vi "UHR-Fleezers Control (host) - 10.4.vi"() -> ()   [LabVIEW 2010] (continued)
        n1177 = event-data() -> ()  [unwired: 7 out]
        n1178 = Negate(x="Phase adj. (AI1)") -> (-x=w4472:i16)
        n1179 = Select(t=w4472, s="- phase (AI1)", f="Phase adj. (AI1)") -> (s? t:f=w4471:i16)
        n1180 = xnode "Read/Write Control"("FPGA VI Reference In"=w4475, "error in"=w4474, "Phase count adjustment"=w4471) -> ("FPGA VI Reference Out"=w4470:T20, "error out"=w4469:errorcluster)
        n1181 = Or(x="- phase (AI1)", y="+ phase (AI1)") -> (x .or. y?=w4466:bool)
        n1182 = xnode "Read/Write Control"("FPGA VI Reference In"=w4470, "error in"=w4469, "+ phase"=w4466) -> ("error out"=w4465:errorcluster)  [unwired: 1 out]
      }
      event "Signals to Plot": Double Click {
        w4553 = u32 9868950 ("Color Box")
        n1183 = event-data() -> ("Row"=w4555:i32)  [unwired: 9 out]
        n1184 = property on="All Signals" class="WFChart (strict)"("Active Plot"=w4555) -> (error out=w4566:errorcluster)  [unwired: 2 in, 1 out]
        n1185 = property on="All Signals" class="WFChart (strict)" props=["Plot", "Visible?", "Plot", "Plot Color"](error in=w4566) -> (error out=w4565:errorcluster, "Plot.Visible?"=w4564:bool)  [unwired: 1 in, 2 out]
        n1186 = Select(t=FALSE ("Plot.Visible"), s=w4564, f=TRUE ("Plot.Visible")) -> (s? t:f=w4559:bool)
        n1187 = property on="All Signals" class="WFChart (strict)"(error in=w4565, "Plot.Visible?"=w4559) -> (error out=w4561:errorcluster)  [unwired: 1 in, 1 out]
        n1188 = property on="All Signals" class="WFChart (strict)"(error in=w4561) -> (error out=w4556:errorcluster, "Plot.Plot Color"=w4560:u32)  [unwired: 1 in, 1 out]
        n1189 = property on="Signals to Plot" class="LstBox (strict)"(error in=w4556, "Active Row"=w4555) -> (error out=w4554:errorcluster)  [unwired: 1 in, 1 out]
        n1190 = Select(t=w4560, s=w4559, f=u32 0) -> (s? t:f=w4557:u32)
        n1191 = property on="Signals to Plot" class="LstBox (strict)"(error in=w4554, "CellFontColor"=w4557, "SelColor"=w4553, "CellBG"=w4553, "CellFontSize"=u32 20 ("Active Row:Cell Font:Size"), "CellFontBold"=TRUE ("Active Row:Cell Font:Bold")) -> ()  [unwired: 1 in, 2 out]
      }
      event "BD 1 Frequency 1 (MHz)", "BD 1 Frequency 2 (MHz)", "BD 1 Frequency 3 (MHz)", "BD 2 Frequency 1 (MHz)", "BD 2 Frequency 2 (MHz)", "BD 2 Frequency 3 (MHz)", "Trap Delta (MHz)": Value Change {
        # "anytime one of the frequencies is changed, write it to the RF board UNLESS Set 1 is being oscillated. The oscillation\nscript writes the frequencies to the RF board."
        n1192 = event-data() -> ("CtlRef"=w4569:refnum<vi>)  [unwired: 6 out]
        n1193 = control-ref of="Trap Delta (MHz)"() -> (w4568:refnum<vi>)
        n1194 = Equal?(x=w4568, y=w4569) -> (x = y?=w4567:bool)
        n1195 = case shown="False" "Oscillate Set 1" {
          tunnel: w4572 -> [w4592 _]
          tunnel: [w4591 w4595] -> w4571
          tunnel: w4570 -> [w4590 w4595]
          tunnel: w4567 -> [w4575 _]
          frame False {
            n1196 = local read "BD 1 Frequency 2 (MHz)"() -> (w4579:dbl)
            n1197 = local read "BD 1 Frequency 1 (MHz)"() -> (w4577:dbl)
            n1198 = Subtract(x=w4579, y="Trap Delta (MHz)") -> (x-y=w4576:dbl)
            n1199 = Select(t=w4576, s=w4575, f=w4577) -> (s? t:f=w4574:dbl)
            n1200 = local read "Y RF Frequency Limits (MHz)"() -> (w4580:T17)
            n1201 = local read "X RF Frequency Limits (MHz)"() -> (w4581:T17)
            n1202 = local read "BD 1 Frequency 3 (MHz)"() -> (w4593:dbl)
            n1203 = local write "BD 1 Frequency 1 (MHz)"(w4574) -> ()
            n1204 = local read "BD 2 Frequency 1 (MHz)"() -> (w4584:dbl)
            n1205 = local read "BD 2 Frequency 2 (MHz)"() -> (w4583:dbl)
            n1206 = local read "BD 2 Frequency 3 (MHz)"() -> (w4594:dbl)
            n1207 = call "set RF board frequency - interlace.vi"("Board 2 Frequency Limits"=w4580, "Board 1 Frequency Limits"=w4581, "error in"=w4590, "FPGA VI Reference In"=w4592, "Board 2 Frequency 3 (MHz)"=w4594, "Board 1 Frequency 3 (MHz)"=w4593, "Board 2 Frequency 2 (MHz)"=w4583, "Board 2 Frequency 1 (MHz)"=w4584, "Board 1 Frequency 2 (MHz)"=w4579, "Board 1 Frequency 1  (MHz)"=w4574) -> ("error out"=w4591:errorcluster)  [unwired: 1 out]
            n1208 = Subtract(x=w4584, y=w4583) -> (x-y=w4588:dbl)
            n1209 = Subtract(x=w4574, y=w4579) -> (x-y=w4589:dbl)
            n1210 = Square(x=w4588) -> (x^2=w4586:dbl)
            n1211 = Square(x=w4589) -> (x^2=w4587:dbl)
            n1212 = Add(x=w4587, y=w4586) -> (x+y=w4585:dbl)
            n1213 = Square Root(x=w4585) -> (sqrt(x)=w4582:dbl)
            n1214 = local write "Trap Delta (MHz)"(w4582) -> ()
            n1215 = property on="Initial delta (MHz)" class="DigNum (strict)"("Val(Sgnl)"=w4582) -> ()  [unwired: 2 in, 2 out]
          }
          frame True {
          }
        }
      }
      event "Round T1 X": Value Change {
        n1216 = event-data() -> ()  [unwired: 7 out]
        n1217 = local read "BD 1 Frequency 1 (MHz)"() -> (w4598:dbl)
        n1218 = Round To Nearest(number=w4598) -> (nearest integer value=w4597:dbl)
        n1219 = property on="BD 1 Frequency 1 (MHz)" class="DigNum (strict)"("Val(Sgnl)"=w4597) -> ()  [unwired: 2 in, 2 out]
      }
      event "Round T2 X": Value Change {
        n1220 = event-data() -> ()  [unwired: 7 out]
        n1221 = local read "BD 1 Frequency 2 (MHz)"() -> (w4600:dbl)
        n1222 = Round To Nearest(number=w4600) -> (nearest integer value=w4599:dbl)
        n1223 = property on="BD 1 Frequency 2 (MHz)" class="DigNum (strict)"("Val(Sgnl)"=w4599) -> ()  [unwired: 2 in, 2 out]
      }
      event "Stop All": Value Change {
        n1224 = event-data() -> ()  [unwired: 7 out]
        n1225 = local read "Stop All"() -> (w4602:bool)
      }
      event "Delayed Interlace Start": Value Change {
        n1226 = event-data() -> ()  [unwired: 7 out]
        n1227 = flat-sequence {
          frame #0 {
            n1228 = Multiply(x="Delay to Interlace (s)", y=1000.0) -> (x*y=w4605:dbl)
            n1229 = Wait (ms)(milliseconds to wait=w4605) -> ()  [unwired: 1 out]
          }
          frame #1 {
            n1230 = property on="Green laser mode" class="RadioBtnsControl (strict)"("Val(Sgnl)"=enum32{"Laser ON", "Laser OFF", "Interlace"}."Interlace" ("Value (Signaling)")) -> ()  [unwired: 2 in, 2 out]
          }
        }
      }
      event "BD 1 Amplitude 1 (%)", "BD 1 Amplitude 2 (%)", "BD 1 Amplitude 3 (%)", "BD 2 Amplitude 1 (%)", "BD 2 Amplitude 2 (%)", "BD 2 Amplitude 3 (%)", "Trap 1 ON", "Trap 2 ON", "Trap 3 ON", "Feedback On/Off", "All FB On/Off": Value Change {
        w4629 = i16 1 ("f")
        n1231 = event-data() -> ()  [unwired: 7 out]
        n1232 = local write "Trap 1 (ON/OFF)"("Trap 1 ON") -> ()
        n1233 = local write "Trap 2 (ON/OFF)"("Trap 2 ON") -> ()
        n1234 = Boolean To (0,1)(Boolean="Trap 3 ON") -> (0, 1=w4630:i16)
        n1235 = Boolean To (0,1)(Boolean="Trap 1 ON") -> (0, 1=w4631:i16)
        n1236 = Boolean To (0,1)(Boolean="Trap 2 ON") -> (0, 1=w4632:i16)
        n1237 = Select(t=w4632, s="Trap ON/OFF X or Y Amp?", f=w4629) -> (s? t:f=w4627:i16)
        n1238 = Select(t=w4631, s="Trap ON/OFF X or Y Amp?", f=w4629) -> (s? t:f=w4628:i16)
        n1239 = Select(t=w4630, s="Trap ON/OFF X or Y Amp?", f=w4629) -> (s? t:f=w4626:i16)
        n1240 = Select(t=w4629, s="Trap ON/OFF X or Y Amp?", f=w4632) -> (s? t:f=w4624:i16)
        n1241 = Select(t=w4629, s="Trap ON/OFF X or Y Amp?", f=w4631) -> (s? t:f=w4625:i16)
        n1242 = Select(t=w4629, s="Trap ON/OFF X or Y Amp?", f=w4630) -> (s? t:f=w4623:i16)
        n1243 = And(x="All FB On/Off", y="Feedback On/Off") -> (x .and. y?=w4621:cluster{"Set 1":bool, "Set 2":bool})
        n1244 = local read "BD 1 Amplitude 1 (%)"() -> (w4641:dbl)
        n1245 = local read "BD 1 Amplitude 2 (%)"() -> (w4640:dbl)
        n1246 = local read "BD 1 Amplitude 3 (%)"() -> (w4639:dbl)
        n1247 = Unbundle By Name(w4621) -> ("Set 1"=w4616:bool, "Set 2"=w4613:bool)
        n1248 = local read "Y RF Amplitude Limits (%)"() -> (w4609:T17)
        n1249 = local read "X RF Amplitude Limits (%)"() -> (w4610:T17)
        n1250 = local read "BD 2 Amplitude 1 (%)"() -> (w4642:dbl)
        n1251 = local read "BD 2 Amplitude 2 (%)"() -> (w4643:dbl)
        n1252 = local read "BD 2 Amplitude 3 (%)"() -> (w4644:dbl)
        n1253 = And(x="Trap 2 ON", y=w4613) -> (x .and. y?=w4611:bool)
        n1254 = And(x="Trap 1 ON", y=w4616) -> (x .and. y?=w4614:bool)
        n1255 = Multiply(x=w4628, y=w4641) -> (x*y=w4636:dbl)
        n1256 = Multiply(x=w4640, y=w4627) -> (x*y=w4634:dbl)
        n1257 = Multiply(x=w4639, y=w4626) -> (x*y=w4635:dbl)
        n1258 = Multiply(x=w4642, y=w4625) -> (x*y=w4645:dbl)
        n1259 = Multiply(x=w4643, y=w4624) -> (x*y=w4646:dbl)
        n1260 = Multiply(x=w4644, y=w4623) -> (x*y=w4647:dbl)
        n1261 = call "set RF board amplitude - interlace.vi"("Board 2 Amplitude Limits"=w4609, "Board 1 Amplitude Limits"=w4610, "error in"=w4637, "FPGA VI Reference In"=w4638, "Board 2 Amplitude 3 (%)"=w4647, "Board 1 Amplitude 3 (%)"=w4635, "Board 2 Amplitude 2 (%)"=w4646, "Board 2 Amplitude 1 (%)"=w4645, "Board 1 Amplitude 2 (%)"=w4634, "Board 1 Amplitude 1 (%)"=w4636) -> ("error out"=w4618:errorcluster, "FPGA VI Reference Out"=w4619:T20)
        n1262 = xnode "Read/Write Control"("FPGA VI Reference In"=w4619, "error in"=w4618, "FB On/Off Set 1"=w4614, "FB On/Off Set 2"=w4611) -> ("error out"=w4617:errorcluster)  [unwired: 1 out]
      }
      event "Load parameters": Value Change {
        n1263 = event-data() -> ()  [unwired: 7 out]
        n1264 = property on="Saved AOD Raster Scan Parameter Sets" class="Arr (strict)"() -> ("Index Values"=w4717:u32[])  [unwired: 2 in, 2 out]
        n1265 = Index Array(array=w4717, index=0) -> (element=w4714:u32)
        n1266 = local write "Load parameters"(FALSE ("Load parameters")) -> ()
        n1267 = Index Array(array="Saved AOD Raster Scan Parameter Sets", index=w4714) -> (element=w4713:T46)
        n1268 = Unbundle By Name(w4713) -> ("Scan Range AOD (nm) 2"=w4712:dbl, "Step Size AOD (nm) 2"=w4711:dbl, "Scan Speed AOD (nm/s) 2"=w4710:dbl, "Number of scans (AOD) 2"=w4709:u16)
        n1269 = flat-sequence {
          tunnel: w4712 -> [w4720]
          tunnel: w4711 -> [w4719]
          tunnel: w4710 -> [w4718]
          tunnel: w4709 -> [w4721]
          frame #0 {
            n1270 = local write "Scan Speed (nm/s)"(w4718) -> ()
            n1271 = local write "Scan Range (nm)"(w4720) -> ()
            n1272 = local write "Step Size (nm)"(w4719) -> ()
          }
          frame #1 {
            n1273 = property on="Number of F/B Scans (AOD)" class="DigNum (strict)"("Val(Sgnl)"=w4721) -> ()  [unwired: 2 in, 2 out]
          }
        }
      }
      event "Trap 1 (ON/OFF)", "Trap 2 (ON/OFF)": Value Change {
        n1274 = event-data() -> ()  [unwired: 7 out]
        n1275 = property on="Trap 2 ON" class="Bool (strict)"("Val(Sgnl)"="Trap 2 (ON/OFF)") -> ()  [unwired: 2 in, 2 out]
        n1276 = property on="Trap 1 ON" class="Bool (strict)"("Val(Sgnl)"="Trap 1 (ON/OFF)") -> ()  [unwired: 2 in, 2 out]
      }
      event "DIO count 1 (ticks)", "DIO count 2 (ticks)", "DIO count 3 (ticks)", "Interlace", "Number Interlace Sets", "Not-Interlacing Set": Value Change {
        n1277 = event-data() -> ()  [unwired: 7 out]
        n1278 = local read "DIO count 3 (ticks)"() -> (w4734:u32)
        n1279 = local read "DIO count 1 (ticks)"() -> (w4736:u32)
        n1280 = local read "DIO count 2 (ticks)"() -> (w4735:u32)
        n1281 = To Unsigned Byte Integer(number="Not-Interlacing Set") -> (unsigned 8bit integer=w4725:u8)
        n1282 = Add(x=w4725, y=u8 1) -> (x+y=w4729:u8)
        n1283 = xnode "Read/Write Control"("FPGA VI Reference In"=w4740, "error in"=w4738, "DIO count 1 (ticks)"=w4736, "DIO count 2 (ticks)"=w4735, "DIO count 3 (ticks)"=w4734, "Interlace ON/OFF"="Interlace", "Number Interlace Cycles"="Number Interlace Sets", "Interlace Off Parameters"=w4729) -> ("error out"=w4739:errorcluster)  [unwired: 1 out]
        n1284 = Build Array(w4736, w4735, w4734) -> (w4727:u32[])
        n1285 = Split 1D Array(array=w4727, index="Number Interlace Sets") -> (first subarray=w4737:u32[])  [unwired: 1 out]
        n1286 = Index Array(array=w4727, index=w4725) -> (element=w4726:u32)
        n1287 = Add Array Elements(numeric array=w4737) -> (sum=w4731:u32)
        n1288 = Select(t=w4731, s="Interlace", f=w4726) -> (s? t:f=→"Total Counts (ticks)":u32)
      }
      event "Reset Feedback": Value Change {
        n1289 = event-data() -> ()  [unwired: 7 out]
        n1290 = Unbundle By Name("Reset Feedback") -> ("Set 1"=w4882:bool, "Set 2"=w4881:bool)
        n1291 = xnode "Read/Write Control"("FPGA VI Reference In"=w4884, "error in"=w4879, "FB Reset Set 1"=w4882, "FB Reset Set 2"=w4881) -> ("error out"=w4880:errorcluster)  [unwired: 1 out]
      }
      event "PID Gains": Value Change {
        n1292 = event-data() -> ()  [unwired: 7 out]
        n1293 = Unbundle By Name("PID Gains") -> ("Set 1"=w4947:T15, "Set 2"=w4946:T15)
        n1294 = xnode "Read/Write Control"("FPGA VI Reference In"=w4948, "error in"=w4944, "FB Gains Set 1"=w4947, "FB Gains Set 2"=w4946) -> ("error out"=w4945:errorcluster)  [unwired: 1 out]
      }
      event "AI2 to Setpoint", "Setpoints (V)": Value Change {
        n1295 = event-data() -> ()  [unwired: 7 out]
        n1296 = xnode "Read/Write Control"("FPGA VI Reference In"=w5023, "error in"=w5019) -> ("FPGA VI Reference Out"=w5022:T20, "error out"=w5021:errorcluster, "AI2 Y Sum Set 1"=w5030:i16, "AI2 Y Sum Set 2"=w5029:i16)
        n1297 = Cluster To Array(cluster="AI2 to Setpoint") -> (array=w5033:bool[])
        n1298 = local read "AI2 (V)"() -> (w5031:cluster{"Set 1":dbl, "Set 2":dbl})
        n1299 = Or Array Elements(Boolean array=w5033) -> (logical OR=w5034:bool)
        n1300 = Bundle By Name(cluster=w5031, "Set 1"=w5030, "Set 2"=w5029) -> (w5028:cluster{"Set 1":dbl, "Set 2":dbl})
        n1301 = Divide(x=w5028, y=3276.7) -> (x/y=w5027:cluster{"Set 1":dbl, "Set 2":dbl})
        "AI2 (V)" <- w5027
        n1302 = case shown="True" w5034 {
          tunnel: [w5098 w5115] -> w5026
          tunnel: "AI2 to Setpoint" -> [_ w5111]
          tunnel: "Setpoints (V)" -> [w5099 w5114]
          tunnel: w5027 -> [_ w5108]
          frame False {
            n1303 = Multiply(x=3276.7, y=w5099) -> (x*y=w5100:cluster{"Set 1":dbl, "Set 2":dbl})
            n1304 = To Word Integer(number=w5100) -> (16bit integer=w5098:cluster{"Set 1":i16, "Set 2":i16})
          }
          frame True {
            n1305 = Unbundle By Name(w5108) -> ("Set 1"=w5107:dbl, "Set 2"=w5106:dbl)
            n1306 = Unbundle By Name(w5114) -> ("Set 1"=w5113:dbl, "Set 2"=w5112:dbl)
            n1307 = Unbundle By Name(w5111) -> ("Set 1"=w5110:bool, "Set 2"=w5109:bool)
            n1308 = Select(t=w5107, s=w5110, f=w5113) -> (s? t:f=w5105:dbl)
            n1309 = Select(t=w5106, s=w5109, f=w5112) -> (s? t:f=w5104:dbl)
            n1310 = Bundle By Name(cluster=w5114, "Set 1"=w5105, "Set 2"=w5104) -> (w5102:cluster{"Set 1":dbl, "Set 2":dbl})
            n1311 = local write "Setpoints (V)"(w5102) -> ()
            n1312 = Multiply(x=3276.7, y=w5102) -> (x*y=w5103:cluster{"Set 1":dbl, "Set 2":dbl})
            n1313 = To Word Integer(number=w5103) -> (16bit integer=w5115:cluster{"Set 1":i16, "Set 2":i16})
          }
        }
        n1314 = Unbundle By Name(w5026) -> ("Set 1"=w5025:i16, "Set 2"=w5024:i16)
        n1315 = xnode "Read/Write Control"("FPGA VI Reference In"=w5022, "error in"=w5021, "FB Setpoint Set 1"=w5025, "FB Setpoint Set 2"=w5024) -> ("error out"=w5020:errorcluster)  [unwired: 1 out]
      }
      event "Invert GI": Value Change {
        n1316 = event-data() -> ()  [unwired: 7 out]
        n1317 = xnode "Read/Write Control"("FPGA VI Reference In"=w5177, "error in"=w5175, "Invert GI"="Invert GI", "Invert GI 2"="Invert GI") -> ("error out"=w5176:errorcluster)  [unwired: 1 out]
      }
      event "Green FB Setpoint (mV)", "Green FB Gains", "Green FB On/Off", "Current When FB OFF (%)", "Green int current ON count adj": Value Change {
        n1318 = event-data() -> ()  [unwired: 7 out]
        n1319 = local read "Green FB Setpoint (mV)"() -> (w5243:dbl)
        n1320 = local read "Current When FB OFF (%)"() -> (w5246:dbl)
        n1321 = Multiply(x=w5243, y=3.2767) -> (x*y=w5242:dbl)
        n1322 = Multiply(x=w5246, y=655.35) -> (x*y=w5247:dbl)
        n1323 = To Unsigned Word Integer(number=w5247) -> (unsigned 16bit integer=w5245:u16)
        n1324 = local read "Green int current ON count adj"() -> (w5250:u32)
        n1325 = local read "Green FB Gains"() -> (w5249:T15)
        n1326 = local read "Green Laser ON/Interlacing"() -> (w5240:bool)
        n1327 = local read "Green laser mode"() -> (w5239:enum32{"Laser ON", "Laser OFF", "Interlace"})
        n1328 = local read "Green FB On/Off"() -> (w5251:bool)
        n1329 = Equal?(x=w5239, y=enum32{"Laser ON", "Laser OFF", "Interlace"}."Interlace") -> (x = y?=w5237:bool)
        n1330 = Compound Arithmetic op=AND(w5237, w5251, w5240) -> (w5241:bool)
        n1331 = xnode "Read/Write Control"("FPGA VI Reference In"=w5254, "error in"=w5253, "Green FB Setpoint"=w5242, "Green FB On/Off"=w5241, "Current Out"=w5245, "Green int current ON count adj"=w5250, "Green FB Gains"=w5249) -> ("error out"=w5252:errorcluster)  [unwired: 1 out]
      }
      event "Green laser mode", "Green Laser ON/Interlacing": Value Change {
        n1332 = event-data() -> ()  [unwired: 7 out]
        n1333 = case shown="True" "Green Laser ON/Interlacing" {
          tunnel: "Green laser mode" -> [_ w5392]
          tunnel: [enum32{"Laser ON", "Laser OFF", "Interlace"}."Laser OFF" ("Green laser mode") w5392] -> w5380
          tunnel: [FALSE w5388] -> w5379
          frame False {
          }
          frame True {
            n1334 = local read "Green FB On/Off"() -> (w5389:bool)
            n1335 = Equal?(x=w5392, y=enum32{"Laser ON", "Laser OFF", "Interlace"}."Interlace") -> (x = y?=w5390:bool)
            n1336 = And(x=w5390, y=w5389) -> (x .and. y?=w5388:bool)
          }
        }
        n1337 = xnode "Read/Write Control"("FPGA VI Reference In"=w5385, "error in"=w5383, "Operating Mode"=w5380, "Operating Mode 2"=w5380, "Green FB On/Off"=w5379) -> ("error out"=w5384:errorcluster)  [unwired: 1 out]
      }
      event "- phase (APD 1 Gate)", "+ phase (APD 1 Gate)": Value Change {
        n1338 = event-data() -> ()  [unwired: 7 out]
        n1339 = local read "Phase Adj. (APD 1 Gate)"() -> (w5471:i16)
        n1340 = Negate(x=w5471) -> (-x=w5479:i16)
        n1341 = Select(t=w5479, s="- phase (APD 1 Gate)", f=w5471) -> (s? t:f=w5478:i16)
        n1342 = Or(x="- phase (APD 1 Gate)", y="+ phase (APD 1 Gate)") -> (x .or. y?=w5474:bool)
        n1343 = xnode "Read/Write Control"("FPGA VI Reference In"=w5481, "error in"=w5480, "Phase count adjustment (APD 1 Gate)"=w5478) -> ("FPGA VI Reference Out"=w5476:T20, "error out"=w5477:errorcluster)
        n1344 = xnode "Read/Write Control"("FPGA VI Reference In"=w5476, "error in"=w5477, "+ phase (APD 1 Gate)"=w5474) -> ("error out"=w5475:errorcluster)  [unwired: 1 out]
      }
      event "+ phase (APD 2 Gate)", "- phase (APD 2 Gate)": Value Change {
        n1345 = event-data() -> ()  [unwired: 7 out]
        n1346 = local read "Phase Adj. (APD 2 Gate)"() -> (w5557:i16)
        n1347 = Negate(x=w5557) -> (-x=w5565:i16)
        n1348 = Select(t=w5565, s="- phase (APD 2 Gate)", f=w5557) -> (s? t:f=w5564:i16)
        n1349 = Or(x="- phase (APD 2 Gate)", y="+ phase (APD 2 Gate)") -> (x .or. y?=w5560:bool)
        n1350 = xnode "Read/Write Control"("FPGA VI Reference In"=w5567, "error in"=w5566, "Phase count adjustment (APD 2 Gate)"=w5564) -> ("FPGA VI Reference Out"=w5562:T20, "error out"=w5563:errorcluster)
        n1351 = xnode "Read/Write Control"("FPGA VI Reference In"=w5562, "error in"=w5563, "+ phase (APD 2 Gate)"=w5560) -> ("error out"=w5561:errorcluster)  [unwired: 1 out]
      }
      event "Phase Adj. (APD Acq)", "+ phase (APD Acq)", "- phase (APD Acq)": Value Change {
        n1352 = event-data() -> ()  [unwired: 7 out]
        n1353 = local read "Phase Adj. (APD Acq)"() -> (w5645:i16)
        n1354 = Negate(x=w5645) -> (-x=w5651:i16)
        n1355 = Select(t=w5651, s="+ phase (APD Acq)", f=w5645) -> (s? t:f=w5650:i16)
        n1356 = Or(x="+ phase (APD Acq)", y="- phase (APD Acq)") -> (x .or. y?=w5646:bool)
        n1357 = xnode "Read/Write Control"("FPGA VI Reference In"=w5653, "error in"=w5652, "Phase Count Adjustment (APD Acq)"=w5650) -> ("FPGA VI Reference Out"=w5648:T20, "error out"=w5649:errorcluster)
        n1358 = xnode "Read/Write Control"("FPGA VI Reference In"=w5648, "error in"=w5649, "+ phase (APD Acq)"=w5646) -> ("error out"=w5647:errorcluster)  [unwired: 1 out]
      }
      event "Phase adj. (GI)", "+ phase (GI)", "- phase (GI)": Value Change {
        n1359 = event-data() -> ()  [unwired: 7 out]
        n1360 = Negate(x="Phase adj. (GI)") -> (-x=w5737:i16)
        n1361 = Select(t=w5737, s="+ phase (GI)", f="Phase adj. (GI)") -> (s? t:f=w5736:i16)
        n1362 = Or(x="+ phase (GI)", y="- phase (GI)") -> (x .or. y?=w5732:bool)
        n1363 = xnode "Read/Write Control"("FPGA VI Reference In"=w5739, "error in"=w5738, "Phase count adjustment (GI)"=w5736) -> ("FPGA VI Reference Out"=w5734:T20, "error out"=w5735:errorcluster)
        n1364 = xnode "Read/Write Control"("FPGA VI Reference In"=w5734, "error in"=w5735, "+ phase (GI)"=w5732) -> ("error out"=w5733:errorcluster)  [unwired: 1 out]
      }
      event "Phase adj. (GI) 2", "+ phase (GI) 2", "- phase (GI) 2": Value Change {
        n1365 = event-data() -> ()  [unwired: 7 out]
        n1366 = Negate(x="Phase adj. (GI) 2") -> (-x=w5823:i16)
        n1367 = Select(t=w5823, s="+ phase (GI) 2", f="Phase adj. (GI) 2") -> (s? t:f=w5822:i16)
        n1368 = Or(x="+ phase (GI) 2", y="- phase (GI) 2") -> (x .or. y?=w5818:bool)
        n1369 = xnode "Read/Write Control"("FPGA VI Reference In"=w5825, "error in"=w5824, "Phase count adjustment (GI) 2"=w5822) -> ("FPGA VI Reference Out"=w5820:T20, "error out"=w5821:errorcluster)
        n1370 = xnode "Read/Write Control"("FPGA VI Reference In"=w5820, "error in"=w5821, "+ phase (GI) 2"=w5818) -> ("error out"=w5819:errorcluster)  [unwired: 1 out]
      }
      event "Phase adj. (Green FB)", "- phase (Green FB)", "+ phase (Green FB)": Value Change {
        n1371 = event-data() -> ()  [unwired: 7 out]
        n1372 = Negate(x="Phase adj. (Green FB)") -> (-x=w5909:i16)
        n1373 = Select(t=w5909, s="+ phase (Green FB)", f="Phase adj. (Green FB)") -> (s? t:f=w5908:i16)
        n1374 = Or(x="+ phase (Green FB)", y="- phase (Green FB)") -> (x .or. y?=w5904:bool)
        n1375 = xnode "Read/Write Control"("FPGA VI Reference In"=w5911, "error in"=w5910, "Phase count adjustment (Green FB)"=w5908) -> ("FPGA VI Reference Out"=w5906:T20, "error out"=w5907:errorcluster)
        n1376 = xnode "Read/Write Control"("FPGA VI Reference In"=w5906, "error in"=w5907, "+ phase (Green FB)"=w5904) -> ("error out"=w5905:errorcluster)  [unwired: 1 out]
      }
      event "Invert APD Gate", "APD Gate ON Count", "APD Gate OFF Count", "APD Gate", "APD Integration Time (s)", "APD 1 AO Mult.", "APD 2 AO Mult.": Value Change {
        n1377 = event-data() -> ()  [unwired: 7 out]
        n1378 = local read "APD Integration Time (s)"() -> (w5987:dbl)
        n1379 = local read "APD Gate ON Count"() -> (w6000:u32)
        n1380 = local read "APD Gate OFF Count"() -> (w5999:u32)
        n1381 = local read "Invert APD Gate"() -> (w6001:bool)
        n1382 = local read "APD Gate"() -> (w5998:enum32{"ON", "OFF", "Interlace"})
        n1383 = Multiply(x=w5987, y=40000000.0) -> (x*y=w5996:dbl)
        n1384 = Reciprocal(x=w5987) -> (1/x=→"APD Acq Rate (Hz)":dbl)
        n1385 = To Unsigned Long Integer(number=w5996) -> (unsigned 32bit integer=w5995:u32)
        n1386 = local read "DMA Update Period (s)"() -> (w5988:dbl)
        n1387 = Divide(x=w5988, y=w5987) -> (x/y=w5991:dbl)
        n1388 = local read "APD 1 AO Mult."() -> (w5993:i16)
        n1389 = local read "APD 2 AO Mult."() -> (w5992:i16)
        n1390 = Multiply(x=2.0, y=w5991) -> (x*y=w5990:dbl)
        n1391 = local write "APD Samples/FIFO Acq."(w5991) -> ()
        n1392 = local write "APD Elements/DMA read"(w5990) -> ()
        n1393 = xnode "Read/Write Control"("FPGA VI Reference In"=w6004, "error in"=w6003, "Invert APD Gate"=w6001, "APD Gate ON Count"=w6000, "APD Gate OFF Count"=w5999, "APD Acq Rate Count"=w5995, "APD Gate Operating Mode"=w5998, "APD 1 AO scale factor"=w5993, "APD 2 AO scale factor"=w5992) -> ("error out"=w6002:errorcluster)  [unwired: 1 out]
      }
      event "GI Frequency, ON count", "Green FB Count", "GI Frequency, OFF count": Value Change {
        n1394 = event-data() -> ()  [unwired: 7 out]
        n1395 = xnode "Read/Write Control"("FPGA VI Reference In"=w6168, "error in"=w6166, "Green interlace ON count"="GI Frequency, ON count", "Green interlace OFF count"="GI Frequency, OFF count", "Green interlace ON count 2"="GI Frequency, ON count", "Green interlace OFF count 2"="GI Frequency, OFF count", "Green FB Count"="Green FB Count") -> ("error out"=w6167:errorcluster)  [unwired: 1 out]
      }
      event "Number of F/B Scans (AOD)", "Scan Speed (nm/s)", "Scan BD", "Initial delta (MHz)", "Step Size (nm)", "Scan Range (nm)": Value Change {
        w6347 = 123.0  # AOM cal (nm/MHz)
        n1396 = event-data() -> ()  [unwired: 7 out]
        n1397 = local read "BD 1 Frequency 1 (MHz)"() -> (w6330:dbl)
        n1398 = local read "AOM X Cal (nm/MHz)"() -> (w6322:dbl)
        n1399 = local read "X RF Frequency Limits (MHz)"() -> (w6334:T17)
        n1400 = local read "Y RF Frequency Limits (MHz)"() -> (w6331:T17)
        n1401 = local read "BD 2 Frequency 1 (MHz)"() -> (w6336:dbl)
        n1402 = Negate(x="Scan Range (nm)") -> (-x=w6300:dbl)
        n1403 = Divide(x=w6300, y=w6322) -> (x/y=w6304:dbl)
        n1404 = Select(t=w6334, s="Scan BD", f=w6331) -> (s? t:f=w6333:T17)
        n1405 = Select(t=w6330, s="Scan BD", f=w6336) -> (s? t:f=w6335:dbl)
        n1406 = Unbundle By Name(w6333) -> ("Maximum"=w6342:dbl, "Minimum"=w6341:dbl)
        n1407 = Add(x=w6304, y=w6335) -> (x+y=w6339:dbl)
        n1408 = Divide(x=w6300, y="Step Size (nm)") -> (x/y=w6319:dbl)
        n1409 = Divide(x="Step Size (nm)", y=w6322) -> (x/y=w6328:dbl)
        n1410 = Absolute Value(x=w6319) -> (abs(x)=w6303:dbl)
        n1411 = Sign(1:w6300) -> (0:w6301:dbl)
        n1412 = In Range and Coerce(upper limit=w6342, x=w6339, lower limit=w6341) -> (coerced(x)=w6338:dbl, In Range?=w6340:bool)
        n1413 = To Unsigned Quad Integer(1:w6303) -> (0:w6318:u64)
        "Scan steps (AOD)" <- w6318
        n1414 = call "IR AOM freq to word.vi"("Frequency In (MHz)"=w6328) -> ("Frequency Word Out (double)"=w6325:dbl)
        n1415 = Multiply(x=w6301, y=w6325) -> (x*y=w6302:dbl)
        n1416 = Subtract(x=w6339, y=w6338) -> (x-y=w6337:dbl)
        n1417 = To Quad Integer(1:w6302) -> (0:w6324:i64)
        "Incr. int (AOD)" <- w6324
        n1418 = Subtract(x=w6304, y=w6337) -> (x-y=w6323:dbl)
        "Scan Range (MHz)" <- w6323
        n1419 = Select(t=w6304, s=w6340, f=w6323) -> (s? t:f=w6343:dbl)
        n1420 = Multiply(x=w6323, y=w6322) -> (x*y=w6321:dbl)
        n1421 = Decrement(x=w6318) -> (x-1=w6371:u64)
        n1422 = Negate(x=w6321) -> (-x=w6317:dbl)
        n1423 = local write "Scan Range (nm)"(w6317) -> ()
        n1424 = Divide(x=w6343, y=w6371) -> (x/y=w6327:dbl)
        "Scan Increment (MHz)" <- w6327
        n1425 = call "IR AOM freq to word.vi"("Frequency In (MHz)"=w6327) -> ("Frequency Word Out (double)"=w6326:dbl)
        n1426 = Divide(x="Step Size (nm)", y="Scan Speed (nm/s)") -> (x/y=w6314:dbl)
        n1427 = To Quad Integer(1:w6326) -> ()  [unwired: 1 out]
        n1428 = local read "Number Interlace Sets"() -> (w6298:u8)
        n1429 = local read "AI Count (ticks)"() -> (w6299:u32)
        n1430 = local read "Total Counts (ticks)"() -> (w6297:u32)
        n1431 = local read "# Samples/trap"() -> (w6329:u32)
        n1432 = Multiply(x=w6299, y=w6298) -> (x*y=w6296:u32)
        n1433 = Divide(x=w6297, y=w6296) -> (x/y=w6295:dbl)
        n1434 = Select(t=w6330, s="Scan BD", f=w6336) -> (s? t:f=w6368:dbl)
        "Initial freq. (MHz)" <- w6368
        n1435 = Add(x=w6343, y=w6368) -> (x+y=→"Final freq. (MHz)":dbl)
        n1436 = Divide(x=w6297, y=40000000.0) -> (x/y=w6313:dbl)
        n1437 = Divide(x=w6314, y=w6313) -> (x/y=w6312:dbl)
        n1438 = To Unsigned Quad Integer(1:w6312) -> (0:w6287:u64)
        n1439 = Quotient & Remainder(x=w6287, y=u64 2) -> (x-y*floor(x/y)=w6291:u64)  [unwired: 1 out]
        n1440 = Equal?(x=w6291, y=u64 0) -> (x = y?=w6289:bool)
        n1441 = Decrement(x=w6287) -> (x-1=w6288:u64)
        n1442 = Select(t=w6287, s=w6289, f=w6288) -> (s? t:f=w6286:u64)
        "Cycles/step (AOD)" <- w6286
        n1443 = xnode "Read/Write Control"("FPGA VI Reference In"=w6379, "error in"=w6378, "Scan steps"=w6318, "Number of scans"="Number of F/B Scans (AOD)", "Cycles per step"=w6286, "Scan freq.  increment"=w6324, "Scan BD"="Scan BD") -> ("error out"=w6377:errorcluster)  [unwired: 1 out]
        n1444 = Multiply(x=w6318, y=w6286) -> (x*y=w6372:u64)
        n1445 = Multiply(x=w6372, y=u64 2) -> (x*y=w6294:u64)
        n1446 = Multiply(x=w6295, y=w6294) -> (x*y=w6293:dbl)
        "Data points/scan (f/b)" <- w6293
        n1447 = Multiply(x=w6293, y="Number of F/B Scans (AOD)") -> (x*y=w6375:dbl)
        "Data points/scans" <- w6375
        n1448 = Divide(x=w6375, y=w6329) -> (x/y=→"N sets should be saved":dbl)
        n1449 = Multiply(x=w6372, y=w6313) -> (x*y=w6311:dbl)
        "Time/Scan (s) (AOD)" <- w6311
        n1450 = Select(t=w6343, s="Scan BD", f=0.0) -> (s? t:f=w6369:dbl)
        n1451 = Select(t=0.0, s="Scan BD", f=w6343) -> (s? t:f=w6365:dbl)
        n1452 = local read "BD 2 Frequency 2 (MHz)"() -> (w6361:dbl)
        n1453 = local read "BD 1 Frequency 2 (MHz)"() -> (w6364:dbl)
        n1454 = Add(x=w6365, y=w6336) -> (x+y=w6362:dbl)
        n1455 = Add(x=w6330, y=w6369) -> (x+y=w6363:dbl)
        n1456 = Multiply(x=w6311, y=2.0) -> (x*y=w6310:dbl)
        n1457 = Multiply(x=w6310, y="Number of F/B Scans (AOD)") -> (x*y=w6307:dbl)
        n1458 = Divide(x=w6307, y=60.0) -> (x/y=→"Time to Finish All (min)":dbl)
        n1459 = Add(x="Trap 2 Bead Size (nm)", y="Trap 1 Bead Size (nm)") -> (x+y=w6351:dbl)
        n1460 = Divide(x=w6351, y=2.0) -> (x/y=w6345:dbl)
        n1461 = local read "Initial delta (MHz)"() -> (w6348:dbl)
        n1462 = Subtract(x=w6362, y=w6361) -> (x-y=w6359:dbl)
        n1463 = Subtract(x=w6363, y=w6364) -> (x-y=w6360:dbl)
        n1464 = Square(x=w6359) -> (x^2=w6358:dbl)
        n1465 = Square(x=w6360) -> (x^2=w6357:dbl)
        n1466 = Add(x=w6357, y=w6358) -> (x+y=w6356:dbl)
        n1467 = Square Root(x=w6356) -> (sqrt(x)=w6355:dbl)
        "Final delta (MHz)" <- w6355
        n1468 = Multiply(x=w6347, y=w6355) -> (x*y=w6354:dbl)
        n1469 = Multiply(x=w6348, y=w6347) -> (x*y=w6346:dbl)
        n1470 = Subtract(x=w6346, y=w6345) -> (x-y=→"Initial sep (nm)":dbl)
        n1471 = Subtract(x=w6354, y=w6345) -> (x-y=→"Final sep (nm)":dbl)
      }
      event "Freq or Amp switch first", "Swap F1 and F2", "Freq switch delay", "Amp switch delay": Value Change {
        n1472 = event-data() -> ()  [unwired: 7 out]
        n1473 = local read "Freq or Amp switch first"() -> (w6516:bool)
        n1474 = local read "Amp switch delay"() -> (w6517:u16)
        n1475 = local read "Freq switch delay"() -> (w6519:u16)
        n1476 = local read "Swap F1 and F2"() -> (w6518:bool)
        n1477 = xnode "Read/Write Control"("FPGA VI Reference In"=w6522, "error in"=w6521, "Freq switch delay"=w6519, "Swap F1 and F2"=w6518, "Amp switch delay"=w6517, "Freq or Amp switch first"=w6516) -> ("error out"=w6520:errorcluster)  [unwired: 1 out]
      }
      event "Scan steps (MCL)", "Number of scans (MCL)", "Scan Range (V)\n(of steps)", "2D or 1D Scan", "N APD Samp/step", "Fast Scan Dir", "Continuous MCL Scanning", "Scan lines (y)": Value Change {
        w6623 = 32767.0 ("y")
        n1478 = event-data() -> ()  [unwired: 7 out]
        n1479 = Select(t="Scan lines (y)", s="2D or 1D Scan", f="Number of scans (MCL)") -> (s? t:f=w6628:u64)
        n1480 = Decrement(x="Scan steps (MCL)") -> (x-1=w6644:u64)
        n1481 = Divide(x="Scan Range (V)\n(of steps)", y=w6644) -> (x/y=w6643:dbl)
        "Desired Scan Incr (V)" <- w6643
        n1482 = local read "APD Integration Time (s)"() -> (w6636:dbl)
        n1483 = Multiply(x=w6643, y=w6623) -> (x*y=w6652:dbl)
        n1484 = Divide(x=w6652, y=10.0) -> (x/y=w6642:dbl)
        "Desired incr (int)" <- w6642
        n1485 = local read "Update Count (MCL)"() -> (w6648:u32)
        n1486 = Round Toward -Infinity(1:w6642) -> (0:w6651:dbl)
        n1487 = To Word Integer(number=w6651) -> (16bit integer=w6626:i16)
        "Actual Incr. int (MCL)" <- w6626
        n1488 = Multiply(x=w6636, y=40000000.0) -> (x*y=w6649:dbl)
        n1489 = Divide(x=w6649, y=w6648) -> (x/y=w6647:dbl)
        n1490 = Multiply(x=i16 10, y=w6626) -> (x*y=w6624:i16)
        n1491 = Multiply(x="N APD Samp/step", y=w6647) -> (x*y=w6646:dbl)
        "Cycles/step (MCL)" <- w6646
        n1492 = Divide(x=w6624, y=w6623) -> (x/y=→"Actual MCL Inc (V)":dbl)
        n1493 = Multiply(x="N APD Samp/step", y="Scan steps (MCL)") -> (x*y=w6638:dbl)
        n1494 = local read "APD Samples/FIFO Acq."() -> (w6635:dbl)
        n1495 = Multiply(x=w6638, y=u64 2) -> (x*y=w6637:dbl)
        "Data points/scan (f+b)" <- w6637
        n1496 = Multiply(x=w6637, y=w6628) -> (x*y=w6655:dbl)
        "Data points/scans (MCL)" <- w6655
        n1497 = Multiply(x=w6636, y=w6637) -> (x*y=w6629:dbl)
        "Time/f+b scan (s) (MCL)" <- w6629
        n1498 = Divide(x=w6655, y=w6635) -> (x/y=→"N sets should be saved (MCL)":dbl)
        n1499 = Multiply(x=w6629, y=w6628) -> (x*y=→"Total Time (s)":dbl)
        n1500 = Not(x="Fast Scan Dir") -> (.not. x?=w6633:bool)
        n1501 = xnode "Read/Write Control"("FPGA VI Reference In"=w6659, "error in"=w6658, "Scan steps (MCL)"="Scan steps (MCL)", "Number of scans (MCL)"=w6628, "Cycles per step (MCL)"=w6646, "Scan freq.  increment (MCL)"=w6626, "1D or 2D Scan?"="2D or 1D Scan", "MCL Scan Axis"=w6633, "Cont. Scan (MCL)"="Continuous MCL Scanning") -> ("error out"=w6657:errorcluster)  [unwired: 1 out]
      }
      event Key Down {
        n1502 = event-data() -> ("VKey"=w6833:T47)  [unwired: 10 out]
        n1503 = local read "z nudge increment (um)"() -> (w6832:dbl)
        n1504 = case shown="\"F8\"" w6833 {
          tunnel: "lateral step size (mm)" -> [w6836 w6841 w6846 w6854 _ _ _ _ _ _ _ _ _ _ _ _ _ _ _ _ _ _ _ _ _ _ _ _ _ _ _ _ _ _ _ _ _ _ _ _ _ _ _ _ _ _ _ _ _ _ _ _ _ _ _ _]
          tunnel: w6832 -> [_ _ _ _ w6857 w6864 _ _ _ _ _ _ _ _ _ _ _ _ _ _ _ _ _ _ _ _ _ _ _ _ _ _ _ _ _ _ _ _ _ _ _ _ _ _ _ _ _ _ _ _ _ _ _ _ _ _]
          frame "Up" {
            w6838 = 0.0 ("element")
            n1505 = Negate(x=w6836) -> (-x=w6835:dbl)
            n1506 = Build Array(w6838, w6835, w6838) -> (w6837:dbl[])
            n1507 = call "CONEX_FUNCTIONAL_GLOBAL.vi"("Axis"=enum16{"X", "Y", "Z", "XY", "XZ", "YZ", "XYZ"}."Y", "Position"=w6837, "Command"=T23."REL MOVE") -> ()  [unwired: 6 in, 3 out]
          }
          frame "Down" {
            w6843 = 0.0 ("element")
            n1508 = Build Array(w6843, w6841, w6843) -> (w6842:dbl[])
            n1509 = call "CONEX_FUNCTIONAL_GLOBAL.vi"("Axis"=enum16{"X", "Y", "Z", "XY", "XZ", "YZ", "XYZ"}."Y", "Position"=w6842, "Command"=T23."REL MOVE") -> ()  [unwired: 6 in, 3 out]
          }
          frame "Left" {
            w6847 = 0.0 ("element")
            n1510 = Build Array(w6846, w6847, w6847) -> (w6848:dbl[])
            n1511 = call "CONEX_FUNCTIONAL_GLOBAL.vi"("Axis"=enum16{"X", "Y", "Z", "XY", "XZ", "YZ", "XYZ"}."X", "Position"=w6848, "Command"=T23."REL MOVE") -> ()  [unwired: 6 in, 3 out]
          }
          frame "Right" {
            w6852 = 0.0 ("element")
            n1512 = Negate(x=w6854) -> (-x=w6853:dbl)
            n1513 = Build Array(w6853, w6852, w6852) -> (w6851:dbl[])
            n1514 = call "CONEX_FUNCTIONAL_GLOBAL.vi"("Axis"=enum16{"X", "Y", "Z", "XY", "XZ", "YZ", "XYZ"}."X", "Position"=w6851, "Command"=T23."REL MOVE") -> ()  [unwired: 6 in, 3 out]
          }
          frame "PageUp" {
            w6861 = 0.0 ("element")
            n1515 = Divide(x=w6857, y=1000.0) -> (x/y=w6859:dbl)
            n1516 = Build Array(w6861, w6861, w6859) -> (w6860:dbl[])
            n1517 = call "CONEX_FUNCTIONAL_GLOBAL.vi"("Axis"=enum16{"X", "Y", "Z", "XY", "XZ", "YZ", "XYZ"}."Z", "Position"=w6860, "Command"=T23."REL MOVE") -> ()  [unwired: 6 in, 3 out]
          }
          frame "PageDown" {
            w6868 = 0.0 ("element")
            n1518 = Divide(x=w6864, y=-1000.0) -> (x/y=w6866:dbl)
            n1519 = Build Array(w6868, w6868, w6866) -> (w6867:dbl[])
            n1520 = call "CONEX_FUNCTIONAL_GLOBAL.vi"("Axis"=enum16{"X", "Y", "Z", "XY", "XZ", "YZ", "XYZ"}."Z", "Position"=w6867, "Command"=T23."REL MOVE") -> ()  [unwired: 6 in, 3 out]
          }
          frame Default {
          }
          frame "Insert" {
          }
          frame "Delete" {
          }
          frame "Home" {
          }
          frame "End" {
          }
          frame "Escape" {
          }
          frame "Help" {
          }
          frame "Pause" {
          }
          frame "ScrollLock" {
          }
          frame "F1" {
          }
          frame "F2" {
          }
          frame "F3" {
          }
          frame "F4" {
          }
          frame "F5" {
          }
          frame "F6" {
          }
          frame "F7" {
          }
          frame "F8" {
          }
          frame "F9" {
          }
          frame "F10" {
          }
          frame "F11" {
          }
          frame "F12" {
          }
          frame "F13" {
          }
          frame "F14" {
          }
          frame "F15" {
          }
          frame "F16" {
          }
          frame "F17" {
          }
          frame "F18" {
          }
          frame "F19" {
          }
          frame "F20" {
          }
          frame "F21" {
          }
          frame "F22" {
          }
          frame "F23" {
          }
          frame "F24" {
          }
          frame "Play" {
          }
          frame "VolumeUp" {
          }
          frame "VolumeDown" {
          }
          frame "Mute" {
          }
          frame "Two Byte Char" {
          }
          frame "Break" {
          }
          frame "Clear" {
          }
          frame "NumLock" {
          }
          frame "Caps" {
          }
          frame "Opt" {
          }
          frame "Cmd" {
          }
          frame "Alt" {
          }
          frame "Ctrl" {
          }
          frame "Shift" {
          }
          frame "Return" {
          }
          frame "Enter" {
          }
          frame "ASCII" {
          }
        }
      }
      event "Read Cal": Value Change {
        w6872 = 1000.0 ("y")
        n1521 = event-data() -> ()  [unwired: 7 out]
        n1522 = local read "Save file name"() -> (w6897:path)
        n1523 = local write "Read Cal"(FALSE ("Read Cal")) -> ()
        n1524 = Strip Path(path=w6897) -> (stripped path=w6896:path)  [unwired: 1 out]
        n1525 = Path To String(path=w6896) -> (string=w6895:string)
        n1526 = Concatenate Strings(w6895, "\\current.cal" ("string")) -> (w6893:string)
        n1527 = String To Path(string=w6893) -> (path=w6892:path)
        n1528 = Open/Create/Replace File(file path (use dialog)=w6892, operation (0:open)=T37."open", access (0:read/write)=enum16{"read/write", "read-only", "write-only"}."read-only") -> (refnum out=w6900:refnum<file>, error out=w6886:errorcluster)  [unwired: 1 in, 3 out]
        n1529 = Deny Access(4:w6886, 7:w6900) -> (0:w6885:errorcluster, 3:w6891:refnum<file>)  [unwired: 1 out]
        n1530 = Read from Binary File(5:0.0, 8:w6885, 9:T38."big-endian, network order" ("byte order (0:big-endian, network order)"), 10:-1 ("count (1)"), 11:w6891) -> (0:w6884:errorcluster, 2:w6882:dbl[], 3:w6887:refnum<file>)  [unwired: 2 out]
        n1531 = Array To Cluster(array=w6882) -> (cluster=w6881:T48)
        n1532 = Unbundle(w6881) -> ("[0]"=w6880:dbl, "[1]"=w6879:dbl, "[2]"=w6878:dbl, "[3]"=w6877:dbl, "[4]"=w6876:dbl, "[5]"=w6875:dbl)
        n1533 = Close File(refnum=w6887, error in=w6884) -> (error out=→"Read cal error":errorcluster)  [unwired: 1 out]
        n1534 = Multiply(x=w6875, y=w6872) -> (x*y=w6873:dbl)
        n1535 = local write "T2 kappa_x (pN/nm)"(w6877) -> ()
        n1536 = local write "T1 kappa_x (pN/nm)"(w6878) -> ()
        n1537 = local write "T1 alpha_x (nm/V)"(w6880) -> ()
        n1538 = local write "T2 alpha_x (nm/V)"(w6879) -> ()
        n1539 = Multiply(x=w6876, y=w6872) -> (x*y=w6874:dbl)
        n1540 = local write "T1 offset_x (mV)"(w6874) -> ()
        n1541 = local write "T2 offset_x (mV)"(w6873) -> ()
      }
      event "Abort MCL Scan": Value Change {
        n1542 = event-data() -> ()  [unwired: 7 out]
        n1543 = local write "MCL Scanning"(FALSE ("MCL Scanning")) -> ()
        n1544 = xnode "Read/Write Control"("FPGA VI Reference In"=w6905, "error in"=w6904, "Abort scan (MCL)"="Abort MCL Scan") -> ("error out"=w6903:errorcluster)  [unwired: 1 out]
      }
      event "Update Count (MCL)": Value Change {
        n1545 = event-data() -> ()  [unwired: 7 out]
        n1546 = xnode "Read/Write Control"("FPGA VI Reference In"=w6947, "error in"=w6946, "MCL count"="Update Count (MCL)") -> ("error out"=w6945:errorcluster)  [unwired: 1 out]
      }
      event "Phase adjust (MCL)", "+ phase (MCL)", "- phase (MCL)": Value Change {
        n1547 = event-data() -> ()  [unwired: 7 out]
        n1548 = Negate(x="Phase adjust (MCL)") -> (-x=w6993:i16)
        n1549 = Select(t=w6993, s="- phase (MCL)", f="Phase adjust (MCL)") -> (s? t:f=w6991:i16)
        n1550 = Or(x="- phase (MCL)", y="+ phase (MCL)") -> (x .or. y?=w6986:bool)
        n1551 = xnode "Read/Write Control"("FPGA VI Reference In"=w6995, "error in"=w6994, "Phase count adjustment (MCL)"=w6991) -> ("FPGA VI Reference Out"=w6987:T20, "error out"=w6988:errorcluster)
        n1552 = xnode "Read/Write Control"("FPGA VI Reference In"=w6987, "error in"=w6988, "+ phase (MCL)"=w6986) -> ("error out"=w6985:errorcluster)  [unwired: 1 out]
      }
      event "Abort AOD Scan": Value Change {
        n1553 = event-data() -> ()  [unwired: 7 out]
        n1554 = xnode "Read/Write Control"("FPGA VI Reference In"=w7074, "error in"=w7073, "Abort scan"="Abort AOD Scan") -> ("error out"=w7072:errorcluster)  [unwired: 1 out]
      }
      event "Continuous AOD Scanning": Value Change {
        n1555 = event-data() -> ()  [unwired: 7 out]
        n1556 = xnode "Read/Write Control"("FPGA VI Reference In"=w7116, "error in"=w7115, "Cont. Scan"="Continuous AOD Scanning") -> ("error out"=w7114:errorcluster)  [unwired: 1 out]
      }
      event "Index": Value Change {
        n1557 = event-data() -> ()  [unwired: 7 out]
        n1558 = call "Create new save file.vi"("Insert"="", "Ext"=".dat" ("string"), "Index In"="Index") -> ("Path Out"=→"Save file name":path, "Index Out"=w7155:dbl)
        "Save index" <- w7155
        n1559 = local write "Index"(w7155) -> ()
      }
      event "AO1", "AO2": Value Change {
        w7170 = 10.0 ("y")
        w7169 = 32767.0 ("y")
        n1560 = event-data() -> ()  [unwired: 7 out]
        n1561 = local read "AO2"() -> (w7168:dbl)
        n1562 = local read "AO1"() -> (w7165:dbl)
        n1563 = Multiply(x=w7165, y=w7169) -> (x*y=w7164:dbl)
        n1564 = Multiply(x=w7168, y=w7169) -> (x*y=w7167:dbl)
        n1565 = Divide(x=w7164, y=w7170) -> (x/y=w7163:dbl)
        n1566 = Divide(x=w7167, y=w7170) -> (x/y=w7166:dbl)
        n1567 = To Word Integer(number=w7163) -> (16bit integer=w7171:i16)
        n1568 = To Word Integer(number=w7166) -> (16bit integer=w7172:i16)
        n1569 = xnode "Read/Write Control"("FPGA VI Reference In"=w7162, "error in"=w7161, "AO1"=w7171, "AO2"=w7172) -> ("error out"=w7160:errorcluster)  [unwired: 1 out]
      }
      event "Inject Pump 1": Value Change {
        n1570 = local read "Chemyx Syringe Pump Serial Port"() -> (w7230:refnum<visa-resource-name>)
        n1571 = event-data() -> ()  [unwired: 7 out]
        n1572 = local read "Pump write delay (ms)"() -> (w7231:dbl)
        n1573 = case shown="True" "Inject Pump 1" {
          tunnel: w7231 -> [w7238 w7252]
          tunnel: w7230 -> [w7235 w7251]
          frame False {
            n1574 = flat-sequence {
              tunnel: w7235 -> [w7239]
              tunnel: [w7239] -> w7236
              tunnel: w7238 -> [_]
              tunnel: [w7242] -> w7237
              tunnel: w7236 -> [w7242]
              tunnel: w7237 -> [w7243]
              tunnel: [w7243] -> w7233
              tunnel: [w7245] -> w7234
              tunnel: w7233 -> [w7245]
              tunnel: w7234 -> [w7247]
              frame #0 {
                n1575 = call "Write to pump.vi"("string"="enter pump1", "VISA resource name"=w7239) -> ()  [unwired: 1 out]
              }
              frame #1 {
                n1576 = Wait (ms)(milliseconds to wait="Pump pause delay (ms)") -> ()  [unwired: 1 out]
              }
              frame #2 {
                n1577 = call "Write to pump.vi"("string"="stop", "VISA resource name"=w7243) -> ()  [unwired: 1 out]
              }
              frame #3 {
                n1578 = Wait (ms)(milliseconds to wait=u32 500) -> ()  [unwired: 1 out]
              }
              frame #4 {
                n1579 = call "Write to pump.vi"("string"="stop", "VISA resource name"=w7247) -> ()  [unwired: 1 out]
              }
            }
          }
          frame True {
            n1580 = flat-sequence {
              tunnel: w7251 -> [w7261]
              tunnel: w7252 -> [w7256]
              tunnel: w7252 -> [w7263]
              tunnel: w7251 -> [w7264]
              tunnel: [w7264] -> w7249
              tunnel: [w7266] -> w7250
              tunnel: w7249 -> [w7266]
              tunnel: w7250 -> [w7268]
              frame #0 {
                n1581 = local read "All Pump Parameters"() -> (w7255:T6)
                n1582 = Unbundle By Name(w7255) -> ("Pump 1"=w7262:T49)
                n1583 = call "Set pump parameters.vi"("Pump write delay (ms)"=w7256, "Volume (uL)"="Ch 2 Inject Volume (uL)", "Rate (uL/h)"="Ch 1 Inject Rate (ul/h)", "Units"=4.0, "Pump #"=1.0, "Pump Parameters In"=w7262, "VISA resource name"=w7261) -> ("Pump Parameters Out"=w7254:T49)  [unwired: 3 in]
                n1584 = Bundle By Name(cluster=w7255, "Pump 1"=w7254) -> (w7253:T6)
                n1585 = local write "All Pump Parameters"(w7253) -> ()
              }
              frame #1 {
                n1586 = Wait (ms)(milliseconds to wait=w7263) -> ()  [unwired: 1 out]
              }
              frame #2 {
                n1587 = call "Write to pump.vi"("string"="start", "VISA resource name"=w7264) -> ()  [unwired: 1 out]
              }
              frame #3 {
                n1588 = Wait (ms)(milliseconds to wait=u32 500) -> ()  [unwired: 1 out]
              }
              frame #4 {
                n1589 = call "Write to pump.vi"("string"="start", "VISA resource name"=w7268) -> ()  [unwired: 1 out]
              }
            }
          }
        }
      }
      event "Inject Pump 3": Value Change {
        n1590 = event-data() -> ()  [unwired: 7 out]
        n1591 = local read "Pump write delay (ms)"() -> (w7271:dbl)
        n1592 = case shown="False" "Inject Pump 3" {
          tunnel: w7271 -> [w7278 w7292]
          tunnel: "Chemyx Syringe Pump Serial Port" -> [w7275 w7291]
          frame False {
            n1593 = flat-sequence {
              tunnel: w7275 -> [w7279]
              tunnel: [w7279] -> w7276
              tunnel: w7278 -> [_]
              tunnel: [w7282] -> w7277
              tunnel: w7276 -> [w7282]
              tunnel: w7277 -> [w7283]
              tunnel: [w7283] -> w7273
              tunnel: [w7285] -> w7274
              tunnel: w7273 -> [w7285]
              tunnel: w7274 -> [w7287]
              frame #0 {
                n1594 = call "Write to pump.vi"("string"="enter pump3", "VISA resource name"=w7279) -> ()  [unwired: 1 out]
              }
              frame #1 {
                n1595 = local read "Pump pause delay (ms)"() -> (w7281:u32)
                n1596 = Wait (ms)(milliseconds to wait=w7281) -> ()  [unwired: 1 out]
              }
              frame #2 {
                n1597 = call "Write to pump.vi"("string"="stop", "VISA resource name"=w7283) -> ()  [unwired: 1 out]
              }
              frame #3 {
                n1598 = Wait (ms)(milliseconds to wait=u32 0) -> ()  [unwired: 1 out]
              }
              frame #4 {
                n1599 = call "Write to pump.vi"("string"="stop", "VISA resource name"=w7287) -> ()  [unwired: 1 out]
              }
            }
          }
          frame True {
            n1600 = flat-sequence {
              tunnel: w7291 -> [w7301]
              tunnel: w7292 -> [w7296]
              tunnel: w7292 -> [w7303]
              tunnel: w7291 -> [w7304]
              tunnel: [w7304] -> w7289
              tunnel: [w7307] -> w7290
              tunnel: w7289 -> [w7307]
              tunnel: w7290 -> [w7308]
              frame #0 {
                n1601 = local read "All Pump Parameters"() -> (w7295:T6)
                n1602 = Unbundle By Name(w7295) -> ("Pump 3"=w7302:T49)
                n1603 = call "Set pump parameters.vi"("Pump write delay (ms)"=w7296, "Volume (uL)"="Ch 3 Inject Volume (uL)", "Rate (uL/h)"="Ch 3 Inject Rate (ul/h)", "Units"=4.0, "Pump #"=3.0, "Pump Parameters In"=w7302, "VISA resource name"=w7301) -> ("Pump Parameters Out"=w7294:T49)  [unwired: 3 in]
                n1604 = Bundle By Name(cluster=w7295, "Pump 3"=w7294) -> (w7293:T6)
                n1605 = local write "All Pump Parameters"(w7293) -> ()
              }
              frame #1 {
                n1606 = Wait (ms)(milliseconds to wait=w7303) -> ()  [unwired: 1 out]
              }
              frame #2 {
                n1607 = call "Write to pump.vi"("string"="start", "VISA resource name"=w7304) -> ()  [unwired: 1 out]
              }
              frame #3 {
                n1608 = Wait (ms)(milliseconds to wait=u32 500) -> ()  [unwired: 1 out]